vi "UHR-Fleezers Control (host) - 10.4.vi"() -> ()   [LabVIEW 2010] (continued)
      }
    }
    n730 = Subtract(x=w1029, y=w1028) -> (x-y=w1027:dbl[])
    n731 = Unbundle By Name(w1062) -> ("Y"=w997:dbl[])
    n732 = Unbundle By Name(w1063) -> ("Y"=w998:dbl[])
    n733 = Build Array(w1063, w1041) -> (→"Force":waveform(dbl)[])
    n734 = Subtract(x=w1027, y="Offset (nm)") -> (x-y=w995:dbl[])
    n735 = call <vilib>:"Mean.vi"("X"=w997) -> ("mean"=w976:dbl)  [unwired: 1 out]
    "T2 X" <- w976
    n736 = Absolute Value(x=w998) -> (abs(x)=w999:dbl[])
    n737 = Absolute Value(x=w997) -> (abs(x)=w1000:dbl[])
    n738 = call <vilib>:"Mean.vi"("X"=w998) -> ("mean"=w977:dbl)  [unwired: 1 out]
    "T1 X" <- w977
    n739 = Add(x=w999, y=w1000) -> (x+y=w1001:dbl[])
    n740 = Bundle By Name(cluster=w1033, "Y"=w995) -> (w963:waveform(dbl))
    "Bead Separation" <- w963
    n741 = Divide(x=w1001, y=2.0) -> (x/y=→"Vec Mean of T1 T2":dbl[])
    n742 = case shown="True" w1010 {
      tunnel: w1052 -> [_ w1927]
      tunnel: w1051 -> [_ w1926]
      tunnel: w1050 -> [_ w1925]
      tunnel: w1047 -> [_ w1924]
      tunnel: w972 -> [_ w1923]
      frame False {
      }
      frame True {
        n743 = property on="Force" class="WFChart (strict)"("YScale.NameLbl.Text"=w1927) -> ()  [unwired: 2 in, 2 out]
        n744 = property on="T2 X" class="DigNum (strict)"("Caption.Text"=w1925) -> ()  [unwired: 2 in, 2 out]
        n745 = property on="T1 X" class="DigNum (strict)"("Caption.Text"=w1926) -> ()  [unwired: 2 in, 2 out]
        n746 = property on="Mean" class="DigNum (strict)"("Caption.Text"=w1924) -> ()  [unwired: 2 in, 2 out]
        n747 = property on="Difference" class="DigNum (strict)"("Caption.Text"=w1923) -> ()  [unwired: 2 in, 2 out]
      }
    }
    n748 = local read "Tether"() -> (w1004:bool)
    n749 = Absolute Value(x=w977) -> (abs(x)=w974:dbl)
    n750 = Absolute Value(x=w976) -> (abs(x)=w973:dbl)
    n751 = Add(x=w974, y=w973) -> (x+y=w1049:dbl)
    n752 = Subtract(x=w974, y=w973) -> (x-y=→"Difference":dbl)
    n753 = feedback #18(w995) -> (w994:dbl[])
    n754 = Divide(x=w1049, y=2.0) -> (x/y=w1003:dbl)
    "Mean" <- w1003
    n755 = case shown="True" w1004 {
      tunnel: w1003 -> [_ w1468]
      frame False {
      }
      frame True {
        n756 = Greater?(x="Lost Tether Alarm Threshold (pN)", y=w1468) -> (0:w1466:bool)
        n757 = case shown="True" w1466 {
          frame False {
          }
          frame True {
            n758 = flat-sequence {
              frame #0 {
                # "stop only if saving"
                n759 = local read "Saving..."() -> (w1481:bool)
                n760 = And(x=w1481, y="TA Cancel Save?") -> (x .and. y?=w1480:bool)
                n761 = local write "Stop Saving"(w1480) -> ()
              }
              frame #1 {
                n762 = case shown="True" "TA Green Off?" {
                  frame False {
                  }
                  frame True {
                    w1484 = FALSE ("Fl. Triggered...")
                    n763 = local write "Fl. Triggered..."(w1484) -> ()
                    n764 = property on="Green Laser ON/Interlacing" class="Bool (strict)"("Val(Sgnl)"=w1484) -> ()  [unwired: 2 in, 2 out]
                  }
                }
              }
            }
            n765 = local read "Time tether formed"() -> (w1475:timestamp)
            n766 = Get Date/Time In Seconds() -> (seconds since 1Jan1904=w1476:timestamp)
            n767 = Subtract(x=w1476, y=w1475) -> (x-y=w1474:dbl)
            n768 = Number To Decimal String(number=w1474) -> (decimal integer string=w1471:string)  [unwired: 1 out]
            n769 = local read "Messages"() -> (w1478:string)
            n770 = call <vilib>:"Beep.vi"() -> ()  [unwired: 3 in, 9 out]
            n771 = Concatenate Strings("Lost tether (" ("Message to add"), w1471, " s)." ("string")) -> (w1473:string)
            n772 = local write "Tether"(FALSE ("Tether")) -> ()
            n773 = call "Update messages.vi"("Message to add"=w1473, "Old message string"=w1478) -> ("New message string"=w1477:string)
            n774 = local write "Messages"(w1477) -> ()
            n775 = property on="Trap Pos. FB ON" class="Bool (strict)"("Val(Sgnl)"=FALSE ("Value (Signaling)")) -> ()  [unwired: 2 in, 2 out]
          }
        }
      }
    }
    n776 = Build Array (concatenate)(w995, w994) -> (w993:dbl[])
    n777 = Split 1D Array(array=w993, index=w875) -> (first subarray=w989:dbl[])  [unwired: 1 out]
    n778 = feedback-in #18(w989) -> ()
    n779 = call <vilib>:"Mean.vi"("X"=w989) -> ("mean"=w988:dbl)  [unwired: 1 out]
    "Bead Mean (nm)" <- w988
    n780 = Subtract(x=w989, y=w988) -> (x-y=w987:dbl[])
    n781 = Square(x=w987) -> (x^2=w986:dbl[])
    n782 = call <vilib>:"Mean.vi"("X"=w986) -> ("mean"=w985:dbl)  [unwired: 1 out]
    n783 = Square Root(x=w985) -> (sqrt(x)=w984:dbl)
    n784 = Multiply(x=10.0, y=w984) -> (x*y=→"RMS (Ang)":dbl)
    n785 = xnode "Read/Write Control"("FPGA VI Reference In"=w1025, "error in"=w1024) -> ("FPGA VI Reference Out"=w1143:T20, "error out"=w1137:errorcluster, "AI2 Y Sum Set 1"=w1133:i16, "AI2 Y Sum Set 2"=w1132:i16, "AI1 X Set 1"=w909:fxp<+/-,16,1>, "AI1 X Set 2"=w908:fxp<+/-,16,1>, "Trap Pos FB Int Signal"=→"Trap Pos FB Int Signal":fxp<+/-,24,9>, "Trap Pos FB Int-Norm Signal"=→"Trap Pos FB Int-Norm Signal":fxp<+/-,16,1>, "Trap Pos FB Action"=w902:i64, "Scanning"=→"AOD Scanning":bool, "Scan I"=→"AOD Scan I":u64, "Scanning MCL"=w1135:bool, "Scan I (MCL)"=→"MCL Scan I":u64, "Green FB Signals"=w1072:T36)  [unwired: 1 out]
    "MCL Scanning" <- w1135
    "Trap Pos FB Action" <- w902
    n786 = local read "AI2 (V)"() -> (w1134:cluster{"Set 1":dbl, "Set 2":dbl})
    n787 = Bundle By Name(cluster=w1134, "Set 1"=w1133, "Set 2"=w1132) -> (w1130:cluster{"Set 1":dbl, "Set 2":dbl})
    n788 = Divide(x=w902, y=327.67) -> (x/y=→"Action (%)":dbl)
    n789 = local read "Trap X (AI1)"() -> (w922:T11)
    n790 = Divide(x=w1130, y=3276.7) -> (x/y=w1129:cluster{"Set 1":dbl, "Set 2":dbl})
    n791 = local write "AI2 (V)"(w1129) -> ()
    n792 = Bundle(cluster=w922, "Trap 1"=w909, "Trap 2"=w908) -> (→"Trap X (AI1)":T11)
    n793 = Divide(x=w1072, y=3276.7) -> (x/y=w1068:T45)
    n794 = Unbundle By Name(w1068) -> ("Green FB Ch 0"=w1071:dbl, "Green FB Ch 1"=w1070:dbl, "Green FB Ch 2"=w1069:dbl)
    n795 = Divide(x=w1071, y=w1069) -> (x/y=w1067:dbl)
    n796 = Divide(x=w1070, y=w1069) -> (x/y=w1066:dbl)
    n797 = flat-sequence "To save data" {
      tunnel: [w3720] -> w1154
      tunnel: [w3721] -> w1153
      tunnel: w1103 -> [w3714]
      tunnel: w991 -> [w3718]
      tunnel: ["Save Calibration"] -> w1126
      tunnel: w1123 -> [w3717]
      tunnel: [w3710] -> w1122
      tunnel: [w3707] -> w1121
      tunnel: [w3704] -> w1120
      tunnel: w1102 -> [w3706]
      tunnel: w1008 -> [w3700]
      tunnel: [w3700] -> w1007
      tunnel: ["Start Saving"] -> w965
      tunnel: [w3694] -> w891
      tunnel: [w3693] -> w890
      tunnel: w1154 -> [w3955]
      tunnel: w1153 -> [w3954]
      tunnel: w892 -> [w3953]
      tunnel: w1126 -> [w3952]
      tunnel: w1122 -> [w3950]
      tunnel: w1121 -> [w3949]
      tunnel: w1120 -> [w3948]
      tunnel: w978 -> [w3947]
      tunnel: w1017 -> [w3946]
      tunnel: w1007 -> [w3945]
      tunnel: w965 -> [w3944]
      tunnel: w963 -> [w3943]
      tunnel: w939 -> [w3942]
      tunnel: w891 -> [w3941]
      tunnel: w890 -> [w3940]
      tunnel: w889 -> [w3939]
      frame #0 {
        n798 = Or(x="Save N Sets", y="Start Saving") -> (x .or. y?=w3701:bool)
        n799 = To Double Precision Float(number=w3717) -> (double precision float=w3711:dbl)
        n800 = Build Array(w3701, "Save Calibration", w3714, w3706) -> (w3716:bool[])
        n801 = Compound Arithmetic op=OR("Save Calibration", w3714, w3701, w3706) -> (w3719:bool)
        n802 = Boolean Array To Number(Boolean array=w3716) -> (number=w3713:u32)
        n803 = feedback #19(FALSE ("Save APD Data\nwith Trap Data")) -> (w3695:bool)
        n804 = feedback #20(refnum<k0> refnum) -> (w3722:refnum<file>)
        n805 = feedback #21(refnum<k0> refnum) -> (w3697:refnum<file>)
        n806 = feedback #22(FALSE ("Save APD Data\nwith Trap Data")) -> (w3705:bool)
        n807 = feedback #23(refnum<k0> refnum) -> (w3708:refnum<file>)
        n808 = feedback #24(0) -> (w3724:i32)
        n809 = feedback #25() -> (w3712:u32)  [unwired: 1 out]
        n810 = case shown="True" w3719 {
          tunnel: [w3731 1] -> w3720
          tunnel: w3724 -> [w3733 _]
          tunnel: [w3732 w3751] -> w3721
          tunnel: w3722 -> [w3732 _]
          tunnel: w3718 -> [_ w3771]
          tunnel: w3711 -> [_ w3769]
          tunnel: w3713 -> [_ w3772]
          tunnel: [w3730 w3750] -> w3710
          tunnel: w3712 -> [w3730 _]
          tunnel: [w3729 w3748] -> w3707
          tunnel: w3708 -> [w3729 _]
          tunnel: [w3728 w3747] -> w3704
          tunnel: w3705 -> [w3728 _]
          tunnel: "Start Saving" -> [_ w3745]
          tunnel: w3700 -> [_ w3744]
          tunnel: [w3727 w3735] -> w3693
          tunnel: w3697 -> [w3727 _]
          tunnel: [w3726 w3734] -> w3694
          tunnel: w3695 -> [w3726 _]
          frame False {
            n811 = Increment(x=w3733) -> (x+1=w3731:i32)
          }
          frame True {
            w3741 = FALSE ("Start Saving")
            w3746 = 9.0  # File Version
            w3754 = FALSE ("prepend array or string size? (T)")
            w3752 = T38."big-endian, network order" ("byte order (0:big-endian, network order)")
            n812 = local read "BD 1 Frequency 1 (MHz)"() -> (w3768:dbl)
            n813 = local read "BD 2 Frequency 1 (MHz)"() -> (w3767:dbl)
            n814 = local read "BD 1 Frequency 2 (MHz)"() -> (w3766:dbl)
            n815 = local read "BD 2 Frequency 2 (MHz)"() -> (w3765:dbl)
            n816 = local read "BD 1 Frequency 3 (MHz)"() -> (w3764:dbl)
            n817 = local read "BD 2 Frequency 3 (MHz)"() -> (w3763:dbl)
            n818 = Array Size(array=w3744) -> (size(s)=w3743:i32)
            n819 = To Double Precision Float(number=w3743) -> (double precision float=w3742:dbl)
            n820 = local write "Save Calibration"(w3741) -> ()
            n821 = local write "Start Saving"(w3741) -> ()
            n822 = Build Array("Save APD Data\nwith Trap Data", "Save Trap Pos. Data") -> (w3738:bool[])
            n823 = Boolean Array To Number(Boolean array=w3738) -> (number=w3737:u32)
            n824 = Build Array(w3768, w3767, w3766, w3765, w3764, w3763) -> (w3762:dbl[])
            n825 = case shown="1, Default" w3772 {
              tunnel: w3771 -> [w3843 w3863 w3879 w3917]
              tunnel: w3742 -> [w3848 w3870 w3899 w3936]
              tunnel: w3769 -> [w3847 w3869 w3898 w3935]
              tunnel: [w3844 w3865 w3890 w3927] -> w3760
              tunnel: [w3835 "Cal sets to save" w3880 w3918] -> w3750
              tunnel: w3762 -> [w3845 w3866 w3892 w3929]
              tunnel: "Save APD Data\nwith Trap Data" -> [w3842 _ w3876 w3915]
              tunnel: [w3842 w3857 w3876 w3915] -> w3747
              tunnel: w3746 -> [w3838 w3858 w3874 w3913]
              tunnel: w3745 -> [w3837 _ _ _]
              tunnel: [w3828 w3857 w3873 w3903] -> w3734
              tunnel: "Save Trap Pos. Data" -> [w3828 _ w3873 w3903]
              tunnel: w3737 -> [w3827 _ w3872 w3902]
              frame 1, Default {
                # "timeseries"
                n826 = case shown="True" "Profile" {
                  tunnel: [w3851 w3854] -> w3832
                  tunnel: [w3851 w3853] -> w3831
                  tunnel: [w3851 w3852] -> w3830
                  tunnel: [w3851 w3856] -> w3829
                  frame False {
                    w3851 = 0.0 ("f")
                  }
                  frame True {
                    n827 = local read "Current Position"() -> (w3855:dbl[])
                    n828 = local read "Y change (mm)"() -> (w3856:dbl)
                    n829 = call "subVI_explode3array.vi"("Array"=w3855) -> ("x"=w3854:dbl, "y"=w3853:dbl, "z"=w3852:dbl)  [unwired: 12 in]
                  }
                }
                n830 = local read "Save ave N"() -> (w3850:dbl)
                n831 = Multiply(x=w3850, y=w3843) -> (x*y=w3849:dbl)
                n832 = To Double Precision Float(number=w3827) -> (double precision float=w3841:dbl)
                n833 = Build Array(w3838, w3843, w3849, w3848, w3847, 0.0 ("f")) -> (w3846:dbl[])
                n834 = Build Array(w3841, w3832, w3831, w3830, w3829) -> (w3839:dbl[])
                n835 = Select(t=u32 4000000000, s=w3837, f="N sets to save") -> (s? t:f=w3835:u32)
                n836 = Build Array (concatenate)(w3846, w3845, w3839) -> (w3844:dbl[])
              }
              frame 2 {
                w3860 = 0.0 ("f")
                w3857 = FALSE ("Save APD Data\nwith Trap Data")
                # "calibration"
                n837 = Boolean To (0,1)(Boolean=w3857) -> (0, 1=w3862:i16)
                n838 = To Double Precision Float(number=w3862) -> (double precision float=w3861:dbl)
                n839 = Build Array(w3861, w3860, w3860, w3860, w3860) -> (w3859:dbl[])
                n840 = Build Array(w3858, w3863, w3863, w3870, w3869, 1.0 ("t")) -> (w3867:dbl[])
                n841 = Build Array (concatenate)(w3867, w3866, w3859) -> (w3865:dbl[])
                "Calibrating Trap..." <- TRUE ("Calibrating...")
              }
              frame 4 {
                w3877 = 0.0 ("f")
                # "scan dir (x/y = 0/1)"
                # "cycles/step"
                # "n scans (f/b)"
                # "steps"
                # "freq. range"
                # "AOD raster scan"
                n842 = local read "Number of F/B Scans (AOD)"() -> (w3884:u16)
                n843 = local read "Cycles/step (AOD)"() -> (w3886:u64)
                n844 = local read "Scan Range (MHz)"() -> (w3889:dbl)
                n845 = local read "Scan steps (AOD)"() -> (w3888:u64)
                n846 = local read "Scan BD"() -> (w3896:bool)
                n847 = local read "Save ave N"() -> (w3901:dbl)
                n848 = Boolean To (0,1)(Boolean=w3896) -> (0, 1=w3895:i16)
                n849 = To Double Precision Float(number=w3884) -> (double precision float=w3883:dbl)
                n850 = To Double Precision Float(number=w3888) -> (double precision float=w3887:dbl)
                n851 = To Double Precision Float(number=w3886) -> (double precision float=w3885:dbl)
                n852 = To Double Precision Float(number=w3895) -> (double precision float=w3894:dbl)
                n853 = Multiply(x=w3901, y=w3879) -> (x*y=w3900:dbl)
                n854 = To Double Precision Float(number=w3872) -> (double precision float=w3878:dbl)
                n855 = Build Array(w3878, w3877, w3877, w3877, w3877) -> (w3875:dbl[])
                n856 = local read "N sets should be saved"() -> (w3881:dbl)
                n857 = Build Array(w3894, w3889, w3887, w3885, w3883) -> (w3891:dbl[])
                n858 = Build Array(w3874, w3879, w3900, w3899, w3898, 2.0 ("t")) -> (w3893:dbl[])
                n859 = Round Toward +Infinity(x=w3881) -> (ceil(x): smallest int >= x=w3882:dbl)
                n860 = Build Array (concatenate)(w3893, w3892, w3875, w3891) -> (w3890:dbl[])
                n861 = To Unsigned Long Integer(number=w3882) -> (unsigned 32bit integer=w3880:u32)
              }
              frame 8 {
                w3910 = 0.0 ("f")
                # "MCL raster scan"
                n862 = local read "Number of scans (MCL)"() -> (w3905:u64)
                n863 = local read "Scan lines (y)"() -> (w3904:u64)
                n864 = local read "2D or 1D Scan"() -> (w3907:bool)
                n865 = local read "Scan Range (V)\n(of steps)"() -> (w3926:dbl)
                n866 = local read "Fast Scan Dir"() -> (w3933:bool)
                n867 = local read "Cycles/step (MCL)"() -> (w3923:u64)
                n868 = local read "Scan steps (MCL)"() -> (w3925:u64)
                n869 = Select(t=w3904, s=w3907, f=w3905) -> (s? t:f=w3906:u64)
                n870 = Boolean To (0,1)(Boolean=w3907) -> (0, 1=w3909:i16)
                n871 = local read "Save ave N"() -> (w3938:dbl)
                n872 = local read "Initial X"() -> (w3912:dbl)
                n873 = local read "Initial Y"() -> (w3911:dbl)
                n874 = To Double Precision Float(number=w3909) -> (double precision float=w3908:dbl)
                n875 = Boolean To (0,1)(Boolean=w3933) -> (0, 1=w3932:i16)
                n876 = To Double Precision Float(number=w3906) -> (double precision float=w3921:dbl)
                n877 = To Double Precision Float(number=w3925) -> (double precision float=w3924:dbl)
                n878 = To Double Precision Float(number=w3923) -> (double precision float=w3922:dbl)
                n879 = To Double Precision Float(number=w3932) -> (double precision float=w3931:dbl)
                n880 = Multiply(x=w3938, y=w3917) -> (x*y=w3937:dbl)
                n881 = To Double Precision Float(number=w3902) -> (double precision float=w3916:dbl)
                n882 = local read "N sets should be saved (MCL)"() -> (w3919:dbl)
                n883 = Build Array(w3916, w3908, w3910, w3910, w3910) -> (w3914:dbl[])
                n884 = Build Array(w3931, w3926, w3924, w3922, w3921, w3912, w3911) -> (w3928:dbl[])
                n885 = Build Array(w3913, w3917, w3937, w3936, w3935, 3.0 ("t")) -> (w3930:dbl[])
                n886 = Round Toward +Infinity(x=w3919) -> (ceil(x): smallest int >= x=w3920:dbl)
                n887 = Build Array (concatenate)(w3930, w3929, w3914, w3928) -> (w3927:dbl[])
                n888 = To Unsigned Long Integer(number=w3920) -> (unsigned 32bit integer=w3918:u32)
              }
            }
            n889 = local read "Index"() -> (w3777:dbl)
            n890 = call "Create new save file.vi"("Insert"="", "Ext"=".dat", "Index In"=w3777) -> ("Path Out"=w3736:path, "Index Out"=w3749:dbl)
            n891 = local write "Save file name"(w3736) -> ()
            n892 = local write "Index"(w3749) -> ()
            n893 = local write "Save index"(w3749) -> ()
            n894 = Array Size(array=w3760) -> (size(s)=w3761:i32)
            n895 = Open/Create/Replace File(file path (use dialog)=w3736, operation (0:open)=T37."create", access (0:read/write)=enum16{"read/write", "read-only", "write-only"}."write-only") -> (refnum out=w3774:refnum<file>)  [unwired: 1 in, 4 out]
            n896 = local write "Saving..."(TRUE ("Saving...")) -> ()
            n897 = To Double Precision Float(number=w3761) -> (double precision float=w3759:dbl)
            n898 = String Length(string="Comment (data description)") -> (length=w3757:i32)
            n899 = To Double Precision Float(number=w3757) -> (double precision float=w3756:dbl)
            n900 = Deny Access(7:w3774) -> (3:w3773:refnum<file>)  [unwired: 1 in, 2 out]
            n901 = Build Array (concatenate)(w3759, w3760, w3756) -> (w3758:dbl[])
            n902 = case "If fluorescence data to be saved" shown="True" w3747 {
              tunnel: w3736 -> [_ w3826]
              tunnel: [refnum<k0> refnum w3806] -> w3748
              frame False {
              }
              frame True {
                w3805 = 0.0
                n903 = local read "APD Integration Time (s)"() -> (w3811:dbl)
                n904 = local read "N APD Samp/step"() -> (w3804:dbl)
                n905 = Path To String(path=w3826) -> (string=w3825:string)
                n906 = String Length(string=w3825) -> (length=w3824:i32)
                n907 = Subtract(x=w3824, y=4) -> (x-y=w3822:i32)
                n908 = String Subset(string=w3825, length (rest)=w3822) -> (substring=w3821:string)  [unwired: 1 out]
                n909 = Build Array(w3811, w3804, w3805, w3805, w3805, w3805, w3805, w3805) -> (w3808:dbl[])
                n910 = Concatenate Strings(w3821, "_fl.dat" ("string")) -> (w3819:string)
                n911 = Array Size(array=w3808) -> (size(s)=w3810:i32)
                n912 = String To Path(string=w3819) -> (path=w3815:path)
                n913 = Open/Create/Replace File(file path (use dialog)=w3815, operation (0:open)=T37."create", access (0:read/write)=enum16{"read/write", "read-only", "write-only"}."write-only") -> (refnum out=w3816:refnum<file>)  [unwired: 1 in, 4 out]
                n914 = Deny Access(7:w3816) -> (3:w3812:refnum<file>)  [unwired: 1 in, 2 out]
                n915 = To Double Precision Float(number=w3810) -> (double precision float=w3809:dbl)
                n916 = Build Array (concatenate)(w3809, w3808) -> (w3807:dbl[])
                n917 = Write to Binary File(file (use dialog)=w3812, data=w3807, 5:FALSE ("prepend array or string size? (T)"), 9:T38."big-endian, network order" ("byte order (0:big-endian, network order)")) -> (refnum out=w3806:refnum<file>)  [unwired: 1 in, 3 out]
              }
            }
            n918 = case shown="True" w3734 {
              tunnel: w3736 -> [_ w3788]
              tunnel: [refnum<k0> refnum w3787] -> w3735
              frame False {
              }
              frame True {
                w3783 = 0.0 ("element")
                n919 = Path To String(path=w3788) -> (string=w3802:string)
                n920 = Build Array(w3783, w3783, w3783, w3783, w3783, w3783, w3783, w3783) -> (w3784:dbl[])
                n921 = String Length(string=w3802) -> (length=w3801:i32)
                n922 = Subtract(x=w3801, y=4) -> (x-y=w3799:i32)
                n923 = Array Size(array=w3784) -> (size(s)=w3786:i32)
                n924 = String Subset(string=w3802, length (rest)=w3799) -> (substring=w3798:string)  [unwired: 1 out]
                n925 = To Double Precision Float(number=w3786) -> (double precision float=w3785:dbl)
                n926 = Concatenate Strings(w3798, "_pos.dat" ("string")) -> (w3796:string)
                n927 = Build Array (concatenate)(w3785, w3784) -> (w3782:dbl[])
                n928 = String To Path(string=w3796) -> (path=w3792:path)
                n929 = Open/Create/Replace File(file path (use dialog)=w3792, operation (0:open)=T37."create", access (0:read/write)=enum16{"read/write", "read-only", "write-only"}."write-only") -> (refnum out=w3793:refnum<file>)  [unwired: 1 in, 4 out]
                n930 = Deny Access(7:w3793) -> (3:w3789:refnum<file>)  [unwired: 1 in, 2 out]
                n931 = Write to Binary File(file (use dialog)=w3789, data=w3782, 5:FALSE ("prepend array or string size? (T)"), 9:T38."big-endian, network order" ("byte order (0:big-endian, network order)")) -> (refnum out=w3787:refnum<file>)  [unwired: 1 in, 3 out]
              }
            }
            n932 = Write to Binary File(file (use dialog)=w3773, data=w3758, 5:w3754, 9:w3752) -> (refnum out=w3755:refnum<file>)  [unwired: 1 in, 3 out]
            n933 = Write to Binary File(file (use dialog)=w3755, data="Comment (data description)", 5:w3754, 9:w3752) -> (refnum out=w3751:refnum<file>)  [unwired: 1 in, 3 out]
          }
        }
        n934 = feedback-in #19(w3694) -> ()
        n935 = feedback-in #20(w3721) -> ()
        n936 = feedback-in #21(w3693) -> ()
        n937 = feedback-in #22(w3704) -> ()
        n938 = feedback-in #23(w3707) -> ()
        n939 = feedback-in #24(w3720) -> ()
        n940 = feedback-in #25(w3710) -> ()
      }
      frame #1 {
        n941 = local read "Saving..."() -> (w3951:bool)
        n942 = case shown="True" w3951 {
          tunnel: w3955 -> [_ w3965]
          tunnel: w3954 -> [_ w3979]
          tunnel: w3953 -> [_ w3975]
          tunnel: w3952 -> [_ w3974]
          tunnel: w3950 -> [_ w3973]
          tunnel: w3949 -> [_ w3968]
          tunnel: w3948 -> [_ w3967]
          tunnel: w3947 -> [_ w3966]
          tunnel: w3946 -> [_ w3964]
          tunnel: w3945 -> [_ w3962]
          tunnel: w3944 -> [_ w3961]
          tunnel: w3943 -> [_ w3960]
          tunnel: w3942 -> [_ w3959]
          tunnel: w3941 -> [_ w3958]
          tunnel: w3940 -> [_ w3957]
          tunnel: w3939 -> [_ w3956]
          frame False {
          }
          frame True {
            n943 = Multiply(x=w3965, y=w3964) -> (x*y=→"Time (s)":dbl)
            n944 = Less Or Equal?(x=w3965, y=w3973) -> (x <= y?=w3977:bool)
            n945 = Or(x="Stop Saving", y="Abort save 2") -> (x .or. y?=w3969:bool)
            n946 = Not(x=w3969) -> (.not. x?=w3978:bool)
            n947 = And(x=w3977, y=w3978) -> (x .and. y?=w3976:bool)
            n948 = case shown="True" w3976 {
              tunnel: w3979 -> [w3986 w4054]
              tunnel: [0.0 w4057] -> w3972
              tunnel: w3965 -> [_ w4055]
              tunnel: w3973 -> [_ w4056]
              tunnel: w3975 -> [_ w4051]
              tunnel: w3974 -> [_ _]
              tunnel: w3968 -> [w3984 w4044]
              tunnel: w3967 -> [w3983 w4045]
              tunnel: w3966 -> [_ w4043]
              tunnel: w3962 -> [_ w4042]
              tunnel: w3961 -> [_ w3996]
              tunnel: w3960 -> [_ w4035]
              tunnel: w3959 -> [_ w4013]
              tunnel: w3958 -> [w3980 w3994]
              tunnel: w3957 -> [w3981 w3993]
              tunnel: w3956 -> [_ w3990]
              frame False {
                w3982 = FALSE
                n949 = Close File(refnum=w3986) -> ()  [unwired: 1 in, 2 out]
                n950 = case shown="True" w3983 {
                  tunnel: w3984 -> [_ w3988]
                  frame False {
                  }
                  frame True {
                    n951 = Close File(refnum=w3988) -> ()  [unwired: 1 in, 2 out]
                  }
                }
                n952 = case shown="True" w3980 {
                  tunnel: w3981 -> [_ w3987]
                  frame False {
                  }
                  frame True {
                    n953 = Close File(refnum=w3987) -> ()  [unwired: 1 in, 2 out]
                  }
                }
                n954 = local write "Raster Scanning..."(w3982) -> ()
                n955 = local write "Calibrating Trap..."(w3982) -> ()
                n956 = call <vilib>:"Beep.vi"() -> ()  [unwired: 3 in, 9 out]
                n957 = local write "Stop Saving"(w3982) -> ()
                "Saving..." <- w3982
              }
              frame True {
                n958 = local read "Calibrating Trap..."() -> (w4046:bool)
                n959 = case "Write fl. data" shown="True" w4045 {
                  tunnel: w4044 -> [_ w4080]
                  tunnel: w4043 -> [_ w4079]
                  frame False {
                  }
                  frame True {
                    n960 = Write to Binary File(file (use dialog)=w4080, data=w4079, 5:FALSE ("prepend array or string size? (T)"), 9:T38."big-endian, network order" ("byte order (0:big-endian, network order)")) -> ()  [unwired: 1 in, 4 out]
                  }
                }
                n961 = Greater?(x="Save ave N", y=1.0) -> (0:w4049:bool)
                n962 = Not(x=w4046) -> (.not. x?=w4048:bool)
                n963 = And(x=w4048, y=w4049) -> (x .and. y?=w3991:bool)
                n964 = case shown="True" w3991 {
                  tunnel: w3990 -> [w4060 w4071]
                  tunnel: [w4060 w4063] -> w3989
                  tunnel: "Save ave N" -> [_ w4064]
                  frame False {
                  }
                  frame True {
                    w4061 = 2 ("dimension size")
                    n965 = Array Size(array=w4071) -> (size(s)=w4065:i32)
                    n966 = Divide(x=w4065, y=w4061) -> (x/y=w4069:dbl)
                    n967 = Reshape Array(w4071, w4069, w4061) -> (w4070:u64[][])
                    n968 = Transpose 2D Array(2D array=w4070) -> (transposed array=w4068:u64[][])
                    n969 = for {
                      tunnel: w4068 -> [w4073] mode=indexing
                      tunnel: [w4072] -> w4062 mode=indexing
                      tunnel: w4064 -> [w4074]
                      workers-P: _ -> [_]
                      n970 = call "downsample 1D array - U64.vi"("Ave N"=w4074, "Array In"=w4073) -> ("Array Out"=w4072:u64[])  [unwired: 1 in]
                    }
                    n971 = Transpose 2D Array(2D array=w4062) -> (transposed array=w4067:u64[][])
                    n972 = Divide(x=w4065, y=w4064) -> (x/y=w4066:dbl)
                    n973 = Reshape Array(w4067, w4066) -> (w4063:u64[])
                  }
                }
                n974 = case shown="True" w3991 {
                  tunnel: w4051 -> [w4083 w4095]
                  tunnel: [w4083 w4087] -> w4047
                  tunnel: "Save ave N" -> [_ w4088]
                  tunnel: w4042 -> [_ w4086]
                  frame False {
                  }
                  frame True {
                    n975 = Array Size(array=w4095) -> (size(s)=w4089:i32)
                    n976 = Array Size(array=w4086) -> (size(s)=w4085:i32)
                    n977 = Divide(x=w4089, y=w4085) -> (x/y=w4093:dbl)
                    n978 = Reshape Array(w4095, w4093, w4085) -> (w4094:i16[][])
                    n979 = Transpose 2D Array(2D array=w4094) -> (transposed array=w4092:i16[][])
                    n980 = for {
                      tunnel: w4092 -> [w4098] mode=indexing
                      tunnel: [w4097] -> w4084 mode=indexing
                      tunnel: w4088 -> [w4096]
                      workers-P: _ -> [_]
                      n981 = call "downsample 1D array - I16.vi"("Ave N"=w4096, "Array In"=w4098) -> ("Array Out"=w4097:i16[])  [unwired: 1 out]
                    }
                    n982 = Transpose 2D Array(2D array=w4084) -> (transposed array=w4091:i16[][])
                    n983 = Divide(x=w4089, y=w4088) -> (x/y=w4090:dbl)
                    n984 = Reshape Array(w4091, w4090) -> (w4087:i16[])
                  }
                }
                n985 = Index Array(array=w4013, index=1) -> (element=w4016:waveform(dbl))
                n986 = Index Array(array=w4013, index=0) -> (element=w4018:waveform(dbl))
                n987 = Unbundle By Name(w4016) -> ("Y"=w4020:dbl[])
                n988 = Unbundle By Name(w4018) -> ("Y"=w4028:dbl[])
                n989 = case "Write trap pos. data" shown="True" w3994 {
                  tunnel: w3993 -> [_ w4076]
                  tunnel: w3989 -> [_ w4075]
                  frame False {
                  }
                  frame True {
                    n990 = Write to Binary File(file (use dialog)=w4076, data=w4075, 5:FALSE ("prepend array or string size? (T)"), 9:T38."big-endian, network order" ("byte order (0:big-endian, network order)")) -> ()  [unwired: 1 in, 4 out]
                  }
                }
                n991 = Write to Binary File(file (use dialog)=w4054, data=w4047, 5:FALSE ("prepend array or string size? (T)"), 9:T38."big-endian, network order" ("byte order (0:big-endian, network order)")) -> ()  [unwired: 1 in, 4 out]
                n992 = feedback #26(w4020) -> (w4022:dbl[])
                n993 = Build Array (concatenate)(w4022, w4020) -> (w4021:dbl[])
                n994 = Select(t=w4020, s=w3996, f=w4021) -> (s? t:f=w4006:dbl[])
                n995 = feedback-in #26(w4006) -> ()
                n996 = feedback #27(w4028) -> (w4041:dbl[])
                n997 = Build Array (concatenate)(w4041, w4028) -> (w4040:dbl[])
                n998 = Select(t=w4028, s=w3996, f=w4040) -> (s? t:f=w4015:dbl[])
                n999 = feedback-in #27(w4015) -> ()
                n1000 = Divide(x=w4055, y=w4056) -> (x/y=w4058:dbl)
                n1001 = Multiply(x=w4058, y=100.0) -> (x*y=w4057:dbl)
                n1002 = Build Array(w4015, w4006) -> (→"Saved APD":dbl[][])
                n1003 = Array Size(array=w4015) -> (size(s)=w4033:i32)
                n1004 = Unbundle By Name(w4035) -> ("Y"=w4039:dbl[])
                n1005 = Subtract(x=w4033, y="N pts to average") -> (x-y=w4009:i32)
                n1006 = Multiply(x="N pts to average", y=u16 2) -> (x*y=w4010:u16)
                n1007 = Subtract(x=w4033, y=w4010) -> (x-y=w4008:i32)
                n1008 = feedback #28(w4039) -> (w4038:dbl[])
                n1009 = Build Array (concatenate)(w4038, w4039) -> (w4037:dbl[])
                n1010 = Select(t=w4039, s=w3996, f=w4037) -> (s? t:f=w4036:dbl[])
                "Trap Delta Graph" <- w4036
                n1011 = feedback-in #28(w4036) -> ()
                n1012 = Array Subset(array=w4015, index=w4009, length="N pts to average") -> (w4032:dbl[])
                n1013 = Array Subset(array=w4015, index=w4008, length="N pts to average") -> (w4031:dbl[])
                n1014 = Array Subset(array=w4006, index=w4009, length="N pts to average") -> (w4012:dbl[])
                n1015 = Array Subset(array=w4006, index=w4008, length="N pts to average") -> (w4011:dbl[])
                n1016 = call <vilib>:"Mean.vi"("X"=w4032) -> ("mean"=w4030:dbl)  [unwired: 1 out]
                n1017 = call <vilib>:"Mean.vi"("X"=w4012) -> ("mean"=w4005:dbl)  [unwired: 1 out]
                n1018 = call <vilib>:"Mean.vi"("X"=w4031) -> ("mean"=w4029:dbl)  [unwired: 1 out]
                n1019 = call <vilib>:"Mean.vi"("X"=w4011) -> ("mean"=w4004:dbl)  [unwired: 1 out]
                n1020 = Subtract(x=w4005, y=w4004) -> (x-y=w3995:dbl)
                "Delta Fl. 2" <- w3995
                n1021 = Subtract(x=w4030, y=w4029) -> (x-y=w4027:dbl)
                "Delta Fl. 1" <- w4027
                n1022 = Initialize Array(w4027, 1 ("dimension size")) -> (w4024:dbl[])
                n1023 = Initialize Array(w3995, 1 ("dimension size")) -> (w4001:dbl[])
                n1024 = feedback #29(w4024) -> (w4025:dbl[])
                n1025 = Build Array (concatenate)(w4025, w4024) -> (w4023:dbl[])
                n1026 = feedback #30(w4001) -> (w4002:dbl[])
                n1027 = Build Array (concatenate)(w4002, w4001) -> (w4000:dbl[])
                n1028 = Select(t=w4024, s=w3996, f=w4023) -> (s? t:f=w3999:dbl[])
                n1029 = feedback-in #29(w3999) -> ()
                n1030 = Select(t=w4001, s=w3996, f=w4000) -> (s? t:f=w3998:dbl[])
                n1031 = feedback-in #30(w3998) -> ()
                n1032 = Build Array(w3999, w3998) -> (→"Save APD Deriv":dbl[][])
              }
            }
            "Progress" <- w3972
            "Progress 2" <- w3972
          }
        }
      }
    }
    n1033 = Bundle By Name(cluster=w1068, "Green FB Ch 0"=w1067, "Green FB Ch 1"=w1066) -> (w1046:T45)
    "Green FB Signals (V)" <- w1046
    n1034 = Unbundle By Name(w1046) -> ("Green FB Ch 2"=→"Green FB Plot":dbl)
    n1035 = local read "wait to reset values"() -> (w1138:bool)
    n1036 = Not(x=w1135) -> (.not. x?=w1139:bool)
    n1037 = And(x=w1139, y=w1138) -> (x .and. y?=w1140:bool)
    n1038 = case "Part of MCL raster scanning: returns to initial positions after scan done" shown="True" w1140 {
      tunnel: w1143 -> [w2689 w2696]
      tunnel: [w2689 w2695] -> w1142
      tunnel: w1137 -> [w2688 w2694]
      tunnel: [w2688 w2693] -> w1136
      frame False {
      }
      frame True {
        w2704 = 10.0 ("y")
        w2703 = 32767.0 ("y")
        # "to return scan values\nafter a synchronous \nAOM scan"
        n1039 = local read "AO2"() -> (w2697:dbl)
        n1040 = local read "AO1"() -> (w2698:dbl)
        n1041 = local write "wait to reset values"(FALSE ("wait to reset values")) -> ()
        n1042 = Multiply(x=w2698, y=w2703) -> (x*y=w2700:dbl)
        n1043 = Multiply(x=w2697, y=w2703) -> (x*y=w2702:dbl)
        n1044 = Divide(x=w2700, y=w2704) -> (x/y=w2699:dbl)
        n1045 = Divide(x=w2702, y=w2704) -> (x/y=w2701:dbl)
        n1046 = To Word Integer(number=w2699) -> (16bit integer=w2705:i16)
        n1047 = To Word Integer(number=w2701) -> (16bit integer=w2706:i16)
        n1048 = local read "Total Counts (ticks)"() -> (w2690:u32)
        n1049 = xnode "Read/Write Control"("FPGA VI Reference In"=w2696, "error in"=w2694, "AO1"=w2705, "AO2"=w2706, "MCL count"=w2690) -> ("FPGA VI Reference Out"=w2695:T20, "error out"=w2693:errorcluster)
        n1050 = local read "Scan Range (V)\n(of steps)"() -> (w2691:dbl)
        n1051 = property on="Scan Range (V)\n(of steps)" class="DigNum (strict)"("Val(Sgnl)"=w2691) -> ()  [unwired: 2 in, 2 out]
      }
    }
    n1052 = node-c288() -> ()  [unwired: 2 out]
  }
  n1053 = node-c288(3 ("Processor")) -> (w63:T25)  [unwired: 3 out]
  n1054 = disable-structure shown="Disabled" {
    disable-tunnel: [w4100 _] -> w218
    disable-tunnel: w18 -> [w4099 _]
    frame Disabled {
      n1055 = node-c288() -> (w4102:T25)  [unwired: 4 out]
      n1056 = timed-loop "Rough control of MCL mirror stage (debugging)" {
        tunnel: w4099 -> [w4105]
        tunnel: [w4104] -> w4100
        timing: w4102 -> [_]
        timing-out: [_] -> w4101
        stop <- w4104 stop-if-true
        n1057 = node-c288() -> ()  [unwired: 2 out]
        n1058 = case shown="1" "MCL Mode" {
          tunnel: w4105 -> [_ w4108 w4212]
          frame 0, Default {
          }
          frame 1 {
            n1059 = node-c288() -> (w4110:T25)  [unwired: 4 out]
            n1060 = timed-loop "Oscillate MCL mirror" {
              timing: w4110 -> [_]
              timing-out: [_] -> w4109
              tunnel: w4108 -> [w4149]
              i -> [w4148]
              stop <- w4111 stop-if-true
              n1061 = node-c288() -> (w4147:i64)  [unwired: 1 out]
              n1062 = Multiply(x="AO1", y=32767.0) -> (x*y=w4143:dbl)
              n1063 = Multiply(x="AO2", y=32767.0) -> (x*y=w4138:dbl)
              n1064 = Divide(x=w4143, y=10.0) -> (x/y=w4144:dbl)
              n1065 = Divide(x=w4138, y=10.0) -> (x/y=w4139:dbl)
              n1066 = To Word Integer(number=w4144) -> (16bit integer=w4136:i16)
              n1067 = To Word Integer(number=w4139) -> (16bit integer=w4135:i16)
              n1068 = Divide(x=w4147, y=i64 1000) -> (x/y=w4118:dbl)
              n1069 = Multiply(x=w4118, y=w4148) -> (x*y=w4129:dbl)
              n1070 = Multiply(x="Osc. freq. (Hz) 2", y=6.283185307179586) -> (x*y=w4130:dbl)
              n1071 = Multiply(x=w4130, y=w4129) -> (x*y=w4128:dbl)
              n1072 = Sine(x=w4128) -> (sin(x)=w4127:dbl)
              n1073 = Multiply(x=w4127, y="Osc. amp. (V)") -> (x*y=w4125:dbl)
              n1074 = Add(x=w4125, y="Osc. center (V)") -> (x+y=w4123:dbl)
              n1075 = Divide(x=w4123, y=10.0) -> (x/y=w4121:dbl)
              n1076 = Multiply(x=w4121, y=32767.0) -> (x*y=w4116:dbl)
              n1077 = Select(t=w4116, s="Scan axis", f=w4136) -> (s? t:f=w4134:dbl)
              n1078 = Select(t=w4135, s="Scan axis", f=w4116) -> (s? t:f=w4133:dbl)
              n1079 = local read "MCL Mode"() -> (w4115:u16)
              n1080 = Not Equal?(x=w4115, y=u16 1) -> (x != y?=w4112:bool)
              n1081 = local read "Stop All"() -> (w4113:bool)
              n1082 = xnode "Read/Write Control"("FPGA VI Reference In"=w4149, "AO1"=w4134, "AO2"=w4133) -> ()  [unwired: 1 in, 2 out]
              n1083 = Compound Arithmetic op=OR(w4113, w4112) -> (w4111:bool)
              n1084 = node-c288() -> ()  [unwired: 2 out]
            }
            n1085 = node-c288(w4109) -> ()  [unwired: 1 out]
          }
          frame 2 {
            n1086 = case shown="True" "Start Scan" {
              tunnel: w4212 -> [_ w4224]
              frame False {
              }
              frame True {
                n1087 = Subtract(x="End (V)", y="Begin (V)") -> (x-y=w4220:dbl)
                n1088 = Decrement(x="N Points") -> (x-1=w4219:dbl)
                n1089 = Divide(x=w4220, y=w4219) -> (x/y=w4217:dbl)
                n1090 = for {
                  N: "N Points" -> [_]
                  tunnel: "Begin (V)" -> [w4237]
                  tunnel: w4224 -> [w4229]
                  tunnel: [w4228] -> w4223 mode=indexing
                  tunnel: w4217 -> [w4227]
                  tunnel: [w4225] -> w4216 mode=indexing
                  i -> [w4236]
                  n1091 = Multiply(x=w4227, y=w4236) -> (x*y=w4235:dbl)
                  n1092 = Add(x=w4237, y=w4235) -> (x+y=w4232:dbl)
                  n1093 = local read "Scan axis"() -> (w4226:bool)
                  n1094 = local read "AO1"() -> (w4234:dbl)
                  n1095 = local read "AO2"() -> (w4233:dbl)
                  n1096 = Select(t=w4232, s=w4226, f=w4234) -> (s? t:f=w4231:dbl)
                  n1097 = Select(t=w4233, s=w4226, f=w4232) -> (s? t:f=w4230:dbl)
                  n1098 = flat-sequence {
                    tunnel: w4231 -> [w4241]
                    tunnel: w4230 -> [w4240]
                    tunnel: w4229 -> [w4238]
                    tunnel: [w4308] -> w4228
                    tunnel: [w4307] -> w4225
                    frame #0 {
                      w4244 = 10.0 ("y")
                      w4239 = 32767.0 ("y")
                      n1099 = Multiply(x=w4241, y=w4239) -> (x*y=w4247:dbl)
                      n1100 = Multiply(x=w4240, y=w4239) -> (x*y=w4245:dbl)
                      n1101 = Divide(x=w4247, y=w4244) -> (x/y=w4248:dbl)
                      n1102 = Divide(x=w4245, y=w4244) -> (x/y=w4246:dbl)
                      n1103 = To Word Integer(number=w4248) -> (16bit integer=w4242:i16)
                      n1104 = To Word Integer(number=w4246) -> (16bit integer=w4243:i16)
                      n1105 = xnode "Read/Write Control"("FPGA VI Reference In"=w4238, "AO1"=w4242, "AO2"=w4243) -> ()  [unwired: 1 in, 2 out]
                    }
                    frame #1 {
                      n1106 = Wait (ms)(milliseconds to wait="DAQ Delay (ms)") -> ()  [unwired: 1 out]
                    }
                    frame #2 {
                      n1107 = local read "Slow mean"() -> (w4308:dbl)
                      n1108 = local read "Sigma"() -> (w4307:dbl)
                    }
                  }
                }
                n1109 = Bundle("Begin (V)"="Begin (V)", w4217, w4223) -> (→"MCL Scan":cluster{"Begin (V)":dbl, dbl, dbl[]})  [unwired: 1 out]
                n1110 = Bundle("Begin (V)"="Begin (V)", w4217, w4216) -> (→"MCL Scan 2":cluster{"Begin (V)":dbl, dbl, dbl[]})  [unwired: 1 out]
              }
            }
          }
        }
        n1111 = local read "Stop All"() -> (w4104:bool)
        n1112 = node-c288() -> ()  [unwired: 2 out]
      }
      n1113 = node-c288(w4101) -> ()  [unwired: 1 out]
    }
    frame Enabled {
    }
  }
  n1114 = timed-loop "Control parameters (event loop)" {
    tunnel: w18 -> [w4315]
    shift-right: [w4314] -> _
    shift-left: errorcluster {"status"=FALSE, "code"=0, "source"=""} ("error out") -> [w4313]
    tunnel: [w4312] -> w216
    timing: w65 -> [_]
    timing-out: [_] -> w64
    tunnel: w42 -> [w4311]
    stop <- w4312 stop-if-true
    n1115 = node-c288() -> ()  [unwired: 2 out]
    n1116 = event shown="[32] Key Down" {
      selector: _ -> [_ _ _ _ _ _ _ _ _ _ _ _ _ _ _ _ _ _ _ _ _ _ _ _ _ _ _ _ _ _ _ _ _ _ _ _ _ _ _ _ _ _ _ _ _ _ _ _ _ _ _ _ _ _]
      dyn-events: _ -> [_ _ _ _ _ _ _ _ _ _ _ _ _ _ _ _ _ _ _ _ _ _ _ _ _ _ _ _ _ _ _ _ _ _ _ _ _ _ _ _ _ _ _ _ _ _ _ _ _ _ _ _ _ _]
      timeout: _ -> [_ _ _ _ _ _ _ _ _ _ _ _ _ _ _ _ _ _ _ _ _ _ _ _ _ _ _ _ _ _ _ _ _ _ _ _ _ _ _ _ _ _ _ _ _ _ _ _ _ _ _ _ _ _]
      tunnel: w4315 -> [w4353 _ _ _ w4475 _ w4572 _ _ _ _ w4638 _ _ w4740 w4884 w4948 w5023 w5177 w5254 w5385 w5481 w5567 w5653 w5739 w5825 w5911 w6004 w6168 w6379 w6522 w6659 _ _ w6905 w6947 w6995 w7074 w7116 _ w7162 _ _ _ _ w7345 _ w7438 w7479 w7526 w7714 w7763 _ w7825]
      tunnel: [w4352 _ _ _ w4465 _ w4571 _ _ w4603 _ w4617 _ _ w4739 w4880 w4945 w5020 w5176 w5252 w5384 w5475 w5561 w5647 w5733 w5819 w5905 w6002 w6167 w6377 w6520 w6657 _ _ w6903 w6945 w6985 w7072 w7114 _ w7160 _ _ _ _ w7343 _ _ _ _ _ _ _ _] -> w4314
      tunnel: w4313 -> [w4351 _ _ _ w4474 _ w4570 _ _ w4603 _ w4637 _ _ w4738 w4879 w4944 w5019 w5175 w5253 w5383 w5480 w5566 w5652 w5738 w5824 w5910 w6003 w6166 w6378 w6521 w6658 _ _ w6904 w6946 w6994 w7073 w7115 _ w7161 _ _ _ _ w7344 _ w7437 w7478 w7525 w7713 w7762 _ w7824]
      tunnel: [_ _ _ _ _ _ _ _ _ w4602 _ _ _ _ _ _ _ _ _ _ _ _ _ _ _ _ _ _ _ _ _ _ _ _ _ _ _ _ _ _ _ _ _ _ _ _ _ _ _ _ _ _ _ _] -> w4312
      tunnel: [_ _ _ _ _ _ _ "Round T1 X" _ _ _ _ _ _ _ _ _ _ _ _ _ _ _ _ _ _ _ _ _ _ _ _ _ _ _ _ _ _ _ _ _ _ _ _ _ _ _ _ _ _ _ _ _ _] -> _
      tunnel: [_ _ _ "Adjust Scale\nto Mean" _ _ _ _ _ _ _ _ _ _ _ _ _ _ _ _ _ _ _ _ _ _ _ _ _ _ _ _ _ _ _ _ _ _ _ _ _ _ _ _ _ _ _ _ _ _ _ "Set SP to Reading" _ _] -> _
      tunnel: [_ _ _ _ _ _ _ _ "Round T2 X" _ "Delayed Interlace Start" _ _ _ _ _ _ _ _ _ _ _ _ _ _ _ _ _ _ _ _ _ _ _ _ _ _ _ _ _ _ _ _ _ _ _ _ _ _ _ _ _ _ _] -> _
      tunnel: w4311 -> [_ _ _ _ _ _ _ _ _ _ _ _ _ _ _ _ _ _ _ _ _ _ _ _ _ _ _ _ _ _ _ _ _ _ _ _ _ _ _ _ _ _ _ _ w7336 _ _ _ _ _ _ _ _ _]
      event "AI Count (ticks)", "Sets to FIFO (Traps)", "Save ave N", "FPGA Ave.", "# Samples/channel", "N sets to save": Value Change {
        # "So that if 'Save ave N' is updated, the AOD scanning code updates too."
        n1117 = event-data() -> ()  [unwired: 6 out]
        n1118 = local read "AI Count (ticks)"() -> (w4333:u32)
        n1119 = Boolean To (0,1)(Boolean="Sets to FIFO (Traps)") -> (0, 1=w4343:cluster{"Set 1":i16, "Set 2":i16, "Set 3":i16})
        n1120 = xnode "Read/Write Control"("FPGA VI Reference In"=w4353, "error in"=w4351, "ai count"=w4333, "AI1 Sets to FIFO"="Sets to FIFO (Traps)", "N of AI1 Int Acq Sets"="N Acq Sets (Traps + Fl.)") -> ("error out"=w4352:errorcluster)  [unwired: 1 out]
        n1121 = Cluster To Array(cluster=w4343) -> (array=w4342:i16[])
        n1122 = To Unsigned Long Integer(number=w4342) -> (unsigned 32bit integer=w4322:u32[])
        n1123 = local read "Scan steps (AOD)"() -> (w4344:u64)
        n1124 = Multiply(x=w4333, y="N Acq Sets (Traps + Fl.)") -> (x*y=w4331:u32)
        n1125 = Divide(x=40000000.0, y=w4333) -> (x/y=w4325:dbl)
        "AI rate (Hz)" <- w4325
        "Ave. Rate (Hz)" <- w4325
        n1126 = Add Array Elements(numeric array=w4322) -> (sum=w4334:u32)
        "Trap Sets" <- w4334
        n1127 = Reciprocal(x=w4325) -> (1/x=→"Ave. Period (s)":dbl)
        n1128 = property on="Scan steps (AOD)" class="DigNum (strict)"("Val(Sgnl)"=w4344) -> ()  [unwired: 2 in, 2 out]
        n1129 = Divide(x=w4325, y="N Acq Sets (Traps + Fl.)") -> (x/y=w4348:dbl)
        "Data Rate (Hz)" <- w4348
        n1130 = Reciprocal(x=w4348) -> (1/x=→"Data Period (s)":dbl)
        n1131 = local read "Save ave N"() -> (w4347:dbl)
        n1132 = Divide(x=w4348, y=w4347) -> (x/y=w4346:dbl)
        "Save Data Rate (Hz)" <- w4346
        n1133 = Reciprocal(x=w4346) -> (1/x=→"Save Data Period (s)":dbl)
        n1134 = Multiply(x=w4331, y="# Samples/trap") -> (x*y=w4329:u32)
        "Counts/DMA" <- w4329
        n1135 = property on="Trap Disp. Downsample" class="DigNum (strict)"("Maximum"="# Samples/trap") -> ()  [unwired: 2 in, 2 out]
        n1136 = Multiply(x=w4334, y="# Samples/trap") -> (x*y=w4323:u32)
        "# Samples/channel" <- w4323
        n1137 = Multiply(x=w4323, y=u32 8) -> (x*y=→"Trap AI Elements/DMA read":u32)
        n1138 = local read "APD Int. Count"() -> (w4330:u32)
        n1139 = Multiply(x=w4323, y=u32 3) -> (x*y=→"Trap Pos Elements/DMA read":u32)
        n1140 = Divide(x=w4329, y=w4330) -> (x/y=w4320:dbl)
        "APD Samples/FIFO Acq." <- w4320
        n1141 = Divide(x=w4329, y=40000000.0) -> (x/y=w4327:dbl)
        "DMA Update Period (s)" <- w4327
        n1142 = Multiply(x=2.0, y=w4320) -> (x*y=→"APD Elements/DMA read":dbl)
        n1143 = property on="APD Disp. Downsample" class="DigNum (strict)"("Maximum"=w4320) -> ()  [unwired: 2 in, 2 out]
        n1144 = local read "N sets to save"() -> (w4340:u32)
        n1145 = Multiply(x=w4327, y=w4340) -> (x*y=→"Total Time (s)":dbl)
        "FPGA Averaging" <- FALSE ("FPGA Averaging")
      }
      event "Rescale on Mean": Value Change {
        n1146 = event-data() -> ()  [unwired: 7 out]
        n1147 = And(x=FALSE, y="Rescale on Mean") -> (x .and. y?=w4440:bool)
        n1148 = local write "Rescale on Mean"(w4440) -> ()
        n1149 = local read "Bead Mean (nm)"() -> (w4445:dbl)
        n1150 = Add(x="Amplitude (nm)", y=w4445) -> (x+y=w4443:dbl)
        n1151 = Subtract(x=w4445, y="Amplitude (nm)") -> (x-y=w4442:dbl)
        n1152 = property on="Bead Separation" class="WFChart (strict)"("YScale.Minimum"=w4442) -> ()  [unwired: 2 in, 2 out]
        n1153 = property on="Bead Separation" class="WFChart (strict)"("YScale.Maximum"=w4443) -> ()  [unwired: 2 in, 2 out]
      }
      event "Detector Type": Value Change {
        n1154 = event-data() -> ()  [unwired: 7 out]
        n1155 = local read "AI labels"() -> (w4446:string[])
        n1156 = property on="High Res. Display" class="Ring (strict)"("Strings []"=w4446) -> ()  [unwired: 2 in, 2 out]
        n1157 = Build Array (concatenate)(w4446, "none") -> (w4447:string[])
        n1158 = property on="FFT 1 Choice 1" class="Ring (strict)"("Strings []"=w4447) -> ()  [unwired: 2 in, 2 out]
        n1159 = property on="FFT 1 Choice 2" class="Ring (strict)"("Strings []"=w4447) -> ()  [unwired: 2 in, 2 out]
        n1160 = property on="FFT 2 Choice 1" class="Ring (strict)"("Strings []"=w4447) -> ()  [unwired: 2 in, 2 out]
        n1161 = property on="FFT 2 Choice 2" class="Ring (strict)"("Strings []"=w4447) -> ()  [unwired: 2 in, 2 out]
        n1162 = Bundle("APD 1", "APD 2") -> (w4450:cluster{string, string})  [unwired: 1 out]
        n1163 = Cluster To Array(cluster=w4450) -> (array=w4448:string[])
        n1164 = Build Array (concatenate)(w4448, w4447) -> (w4452:string[])
        n1165 = Array Size(array=w4452) -> (size(s)=w4453:i32)
        n1166 = property on="Signals to Plot" class="LstBox (strict)"("Item Names"=w4452) -> ()  [unwired: 2 in, 2 out]
        n1167 = property on="Signals to Plot" class="LstBox (strict)"("Number of Rows"=w4453) -> ()  [unwired: 2 in, 2 out]
        n1168 = property on="All Signals" class="WFChart (strict)"("LegNumRows"=w4453) -> ()  [unwired: 2 in, 2 out]
      }
      event "Adjust Scale\nto Mean": Value Change {
        n1169 = event-data() -> ()  [unwired: 7 out]
        n1170 = local read "APD 1 Rate (Hz)"() -> (w4462:dbl)
        n1171 = Multiply(x=1000.0, y="Above (kHz)") -> (x*y=w4460:dbl)
        n1172 = Multiply(x=1000.0, y="Below (kHz)") -> (x*y=w4458:dbl)
        n1173 = Add(x=w4460, y=w4462) -> (x+y=w4455:dbl)
        n1174 = Subtract(x=w4462, y=w4458) -> (x-y=w4456:dbl)
        n1175 = property on="APD Chart" class="WFChart (strict)"("YScale.Minimum"=w4456) -> ()  [unwired: 2 in, 2 out]
        n1176 = property on="APD Chart" class="WFChart (strict)"("YScale.Maximum"=w4455) -> ()  [unwired: 2 in, 2 out]
      }
      event "Phase adj. (AI1)", "+ phase (AI1)", "- phase (AI1)": Value Change {